vi "CRYO_MASTER_FULL_RUN2.vi"() -> ()   [LabVIEW 2017]
uses:
  LSI218Data.lvclass
  LSI336Data.lvclass
  USBData.lvclass
  6240AData.lvclass
  DMMsData.lvclass
  <vilib>/DAQmx/miscellaneous.llb/DAQmx Fill In Error Info.vi
  <vilib>/DAQmx/create/channels.llb/DAQmx Create Channel (DO-Digital Output).vi
  <vilib>/DAQmx/create/channels.llb/DAQmx Create Channel (AO-Voltage-Basic).vi
  <vilib>/express/express arith-compare/Formula/XNode/ExpressFormulaBlockNode.xnode
  <vilib>/Analysis/NI_AALBase.lvlib
  istr.lib/Agilent 33XXX Series/Agilent 33XXX Series.lvlib
panel:
  in  "Automatic \nScreenshots?":bool=TRUE
  in  "Frontpanel screenshots":bool
  in  "Screenshots interval":i64=3605
  in  "Record interval":i64=10
  out "Cycle #":u32=5047
  in  "Measurement Interval (s)":dbl=1.0
  in  "Stop Button":bool
  in  "?":T1(tab)=enum."LSI CONFIG"
  out "RUN Identifier":string="20210201_135757_RUN_III"
  in  "Base Path (screenshots)":path=path "C:/LabVIEW/DATA/Google/TUCAN Experiments/KEK_cryotests_2019-2020/data/screenshots"
  out "error out (USB6210/6218 AOUT)":errorcluster
  in  "AOUT Labels":string[](array[string])=["PWR400H_I", "PMC183A_I"]
  in  "DOUT Labels":string[](array[string])=["D_V1_NO", "D_V2_NC", "D_CV1", "D_H1"]
  in  "AOUT assignment":tag[](array[tag])=["Dev1/ao0", "Dev1/ao1"]
  out "AO task out":refnum<k21>="20210201_135757_RUN_III_AO"
  in  "Analog Out ON?":bool=TRUE
  in  "InstName (USB6218)":string="USB6218"
  in  "USB6218 Config":T2(array[cluster])=[{"Label"="F_1", "FileFormat"="%5.5f", "Active?"=TRUE, "Physical CH"="Dev1/ai0", " terminal\n type"=10083, "ConversionType"={"Type"=enum."SimpleProp", "ConversionParameters"=[0.0, 5.0, 0.0, 500.0]}, "VoltageLimits"=[0.0, 5.0]}, {"Label"="F_2", "FileFormat"="%5.5f", "Active?"=TRUE, "Physical CH"="Dev1/ai1", " terminal\n type"=10083, "ConversionType"={"Type"=enum."SimpleProp", "ConversionParameters"=[0.0, 5.0, 0.0, 200.0]}, "VoltageLimits"=[0.0, 5.0]}, {"Label"="F_3", "FileFormat"="%5.5f", "Active?"=TRUE, "Physical CH"="Dev1/ai2", " terminal\n type"=10083, "ConversionType"={"Type"=enum."SimpleProp", "ConversionParameters"=[0.0, 5.0, 0.0, 200.0]}, "VoltageLimits"=[0.0, 5.0]}, {"Label"="F_4", "FileFormat"="%5.5f", "Active?"=TRUE, "Physical CH"="Dev1/ai3", " terminal\n type"=10083, "ConversionType"={"Type"=enum."SimpleProp", "ConversionParameters"=[0.0, 5.0, 0.0, 500.0]}, "VoltageLimits"=[0.0, 5.0]}, {"Label"="F_5", "FileFormat"="%5.5f", "Active?"=TRUE, "Physical CH"="Dev1/ai4", " terminal\n type"=10083, "ConversionType"={"Type"=enum."SimpleProp", "ConversionParameters"=[0.0, 5.0, 0.0, 500.0]}, "VoltageLimits"=[0.0, 5.0]}, {"Label"="I_CV", "FileFormat"="%3.5f", "Active?"=TRUE, "Physical CH"="Dev1/ai5", " terminal\n type"=10083, "ConversionType"={"Type"=enum."Raw", "ConversionParameters"=[0.0, 0.0, 0.0, 0.0]}, "VoltageLimits"=[0.0, 10.0]}, {"Label"="CV1_answer", "FileFormat"="%3.5f", "Active?"=TRUE, "Physical CH"="Dev1/ai6", " terminal\n type"=10083, "ConversionType"={"Type"=enum."SimpleProp", "ConversionParameters"=[1.0, 5.0, 0.0, 100.0]}, "VoltageLimits"=[0.0, 5.0]}, {"Label"="P_Dewar", "FileFormat"="%5.5e", "Active?"=TRUE, "Physical CH"="Dev1/ai7", " terminal\n type"=10083, "ConversionType"={"Type"=enum."SimpleProp", "ConversionParameters"=[1.0, 5.0, 0.0, 200000.0]}, "VoltageLimits"=[0.0, 5.0]}] {"terminal\n type" items=["Default"=-1, "RSE"=10083, "NRSE"=10078, "Differential"=10106, "Pseudodifferential"=12529]}
  out "error out (USB6218)":errorcluster
  out "error out (USB6210/6218 DOUT)":errorcluster
  out "DOUT task out":refnum<k21>="20210201_135757_DO"
  in  "DOUT Physical CH":tag[](array[tag])=["Dev1/port1/line0", "Dev1/port1/line1", "Dev1/port1/line2", "Dev1/port1/line3"]
  in  "Digital Out ON?":bool=TRUE
  in  "USB6210 Config":T2(array[cluster])=[{"Label"="P_ins", "FileFormat"="%5.5e", "Active?"=TRUE, "Physical CH"="Dev2/ai0", " terminal\n type"=10083, "ConversionType"={"Type"=enum."CC-10_LOG", "ConversionParameters"=[0.5, 9.0, 0.0, 1.0]}, "VoltageLimits"=[0.0, 10.0]}, {"Label"="P_4Kres", "FileFormat"="%5.5e", "Active?"=TRUE, "Physical CH"="Dev2/ai1", " terminal\n type"=10083, "ConversionType"={"Type"=enum."SimpleProp", "ConversionParameters"=[1.0, 5.0, 0.0, 200000.0]}, "VoltageLimits"=[0.0, 5.0]}, {"Label"="P_3HeIN", "FileFormat"="%5.5e", "Active?"=TRUE, "Physical CH"="Dev2/ai2", " terminal\n type"=10083, "ConversionType"={"Type"=enum."SimpleProp", "ConversionParameters"=[1.0, 5.0, 0.0, 200000.0]}, "VoltageLimits"=[0.0, 5.0]}, {"Label"="P_SldRTN", "FileFormat"="%5.5e", "Active?"=TRUE, "Physical CH"="Dev2/ai3", " terminal\n type"=10083, "ConversionType"={"Type"=enum."SimpleProp", "ConversionParameters"=[1.0, 5.0, 0.0, 200000.0]}, "VoltageLimits"=[0.0, 5.0]}, {"Label"="P_3Hepot", "FileFormat"="%5.5e", "Active?"=TRUE, "Physical CH"="Dev2/ai4", " terminal\n type"=10083, "ConversionType"={"Type"=enum."SimpleProp", "ConversionParameters"=[0.0, 10.0, 0.0, 133320.0]}, "VoltageLimits"=[0.0, 10.0]}, {"Label"="P_1Kpot", "FileFormat"="%5.5e", "Active?"=TRUE, "Physical CH"="Dev2/ai5", " terminal\n type"=10083, "ConversionType"={"Type"=enum."SimpleProp", "ConversionParameters"=[0.0, 10.0, 0.0, 133320.0]}, "VoltageLimits"=[0.0, 10.0]}, {"Label"="P_Dewar(old)", "FileFormat"="%5.5e", "Active?"=FALSE, "Physical CH"="Dev2/ai6", " terminal\n type"=10083, "ConversionType"={"Type"=enum."SimpleProp", "ConversionParameters"=[1.0, 5.0, 0.0, 200000.0]}, "VoltageLimits"=[0.0, 5.0]}, {"Label"="DP_HEX4", "FileFormat"="%5.5e", "Active?"=TRUE, "Physical CH"="Dev2/ai7", " terminal\n type"=10083, "ConversionType"={"Type"=enum."SimpleProp", "ConversionParameters"=[1.0, 5.0, 0.0, 1000.0]}, "VoltageLimits"=[0.0, 5.0]}, {"Label"="DP_HEX5", "FileFormat"="%5.5e", "Active?"=TRUE, "Physical CH"="Dev2/ai8", " terminal\n type"=10083, "ConversionType"={"Type"=enum."SimpleProp", "ConversionParameters"=[1.0, 5.0, 0.0, 1000.0]}, "VoltageLimits"=[0.0, 5.0]}, {"Label"="L1", "FileFormat"="%5.5f", "Active?"=TRUE, "Physical CH"="Dev2/ai9", " terminal\n type"=10083, "ConversionType"={"Type"=enum."SimpleProp", "ConversionParameters"=[0.0, 10.0, 0.0, 100.0]}, "VoltageLimits"=[0.0, 10.0]}, {"Label"="L2-1", "FileFormat"="%5.5f", "Active?"=TRUE, "Physical CH"="Dev2/ai10", " terminal\n type"=10083, "ConversionType"={"Type"=enum."SimpleProp", "ConversionParameters"=[0.0, 10.0, 0.0, 100.0]}, "VoltageLimits"=[0.0, 10.0]}, {"Label"="L2-2", "FileFormat"="%5.5f", "Active?"=TRUE, "Physical CH"="Dev2/ai11", " terminal\n type"=10083, "ConversionType"={"Type"=enum."SimpleProp", "ConversionParameters"=[0.0, 10.0, 0.0, 100.0]}, "VoltageLimits"=[0.0, 10.0]}, {"Label"="L3", "FileFormat"="%5.5f", "Active?"=TRUE, "Physical CH"="Dev2/ai12", " terminal\n type"=10083, "ConversionType"={"Type"=enum."SimpleProp", "ConversionParameters"=[0.0, 10.0, 0.0, 100.0]}, "VoltageLimits"=[0.0, 10.0]}, {"Label"="P_HEX7OUT", "FileFormat"="%5.5e", "Active?"=TRUE, "Physical CH"="Dev2/ai13", " terminal\n type"=10083, "ConversionType"={"Type"=enum."SimpleProp", "ConversionParameters"=[1.0, 5.0, 0.0, 200000.0]}, "VoltageLimits"=[0.0, 5.0]}, {"Label"="P_IP", "FileFormat"="%5.5e", "Active?"=TRUE, "Physical CH"="Dev2/ai14", " terminal\n type"=10083, "ConversionType"={"Type"=enum."CC-10_LOG", "ConversionParameters"=[0.5, 9.0, 0.0, 1.0]}, "VoltageLimits"=[0.0, 10.0]}, {"Label"="V_H1", "FileFormat"="%3.5f", "Active?"=TRUE, "Physical CH"="Dev2/ai15", " terminal\n type"=10083, "ConversionType"={"Type"=enum."Raw", "ConversionParameters"=[0.0, 1.0, 0.0, 1.0]}, "VoltageLimits"=[0.0, 10.0]}] {"terminal\n type" items=["Default"=-1, "RSE"=10083, "NRSE"=10078, "Differential"=10106, "Pseudodifferential"=12529]}
  in  "RUN label":string="RUN_III"
  in  "Base Path":path=path "C:/LabVIEW/DATA/RUN_3"
  in  "InstName (USB6210)":string="USB6210"
  out "error out (USB6210)":errorcluster
  out "File Refn USB AO":refnum<file>
  out "File Refn USB DO":refnum<file>
  out "error out (LSI336)":errorcluster
  in  "InstName (LSI336)":string="LSI336"
  in  "FileFormat (336)":string="%4.4f"
  in  "LSI336Settings(X,Y)":T3(array[cluster])=[{"LSIName"="LSi336X", "Labels"=["T1K3-1", "T1K3-2", "T3He5", "T3He8"], "SensorLocations"=[enum."T1K3-1", enum."T1K3-2", enum."T3He5", enum."T3He8"], "Active?"=TRUE, "VISA res. name"="COM15_LSI336Y"}, {"LSIName"="LSi336Y", "Labels"=["T3He6-1", "T3He6-2", "T3He7-1", "T3He7-2"], "SensorLocations"=[enum."T3He6-1", enum."T3He6-2", enum."T3He7-1", enum."T3He7-2"], "Active?"=TRUE, "VISA res. name"="COM20_LSI336X"}]
  in  "FileFormat (218)":string="%4.4f"
  in  "InstName (LSI218)":string="LSI218"
  in  "LSI218Settings(A-F)":T3(array[cluster])=[{"LSIName"="LSI218A", "Labels"=["T3He10", "T3He1-1", "TTH3", "TTH4", "TTH1", "TTH2", "T4He1", "T1K1"], "SensorLocations"=[enum."T3He10", enum."T3He1-1", enum."TTH3", enum."TTH4", enum."TTH1", enum."TTH2", enum."T4He1", enum."T1K1"], "Active?"=TRUE, "VISA res. name"="GPIB0::7::INSTR"}, {"LSIName"="LSI218B", "Labels"=["N.C.", "N.C.", "N.C.", "N.C.", "T3He2-1", "T3He2-2", "T3He3", "T3He1-4"], "SensorLocations"=[enum."N.C.", enum."N.C.", enum."N.C.", enum."N.C.", enum."T3He2-1", enum."T3He2-2", enum."T3He3", enum."T3He1-4"], "Active?"=TRUE, "VISA res. name"="GPIB0::4::INSTR"}, {"LSIName"="LSI218C", "Labels"=["T4He3-1", "T4He3-2", "T4He3-3", "T4He3-4", "T4He2-1", "T4He2-2", "T4He4", "T4He5"], "SensorLocations"=[enum."T4He3-1", enum."T4He3-2", enum."T4He3-3", enum."T4He3-4", enum."T4He2-1", enum."T4He2-2", enum."T4He4", enum."T4He5"], "Active?"=TRUE, "VISA res. name"="GPIB0::3::INSTR"}, {"LSIName"="LSI218D", "Labels"=["T4He6", "T4He9", "T3He1-2", "T3He1-3", "T4He7", "T4He8", "T4He10", "T1K6"], "SensorLocations"=[enum."T4He6", enum."T4He9", enum."T3He1-2", enum."T3He1-3", enum."T4He7", enum."T4He8", enum."T4He10", enum."T1K6"], "Active?"=TRUE, "VISA res. name"="GPIB0::5::INSTR"}, {"LSIName"="LSI218E", "Labels"=["TIP1", "N.C.", "TIP2", "N.C.", "TIP3", "TIP4", "TIP5", "N.C."], "SensorLocations"=[enum."TIP1", enum."N.C.", enum."TIP2", enum."N.C.", enum."TIP3", enum."TIP4", enum."TIP5", enum."N.C."], "Active?"=TRUE, "VISA res. name"="GPIB0::11::INSTR"}, {"LSIName"="LSI218F", "Labels"=["T1K2", "T1K4", "T1K5", "T3He4", "T3He9", "TIP6", "N.C.", "N.C."], "SensorLocations"=[enum."T1K2", enum."T1K4", enum."T1K5", enum."T3He4", enum."T3He9", enum."TIP6", enum."N.C.", enum."N.C."], "Active?"=TRUE, "VISA res. name"="GPIB0::8::INSTR"}]
  out "error out (LSI218)":errorcluster
  out "RUN Identifier 2":string="20210201_135757_RUN_III" caption="RUN Identifier"
  out "Graph 3":T4(graph) caption="XY Graph"
  out "Graph 1":T4(graph) caption="XY Graph"
  in  "FIle suffix 4":string="Graph4_noise"
  in  "Take Screenshot! 4":bool
  in  "Take Screenshot! 3":bool
  in  "Take Screenshot! 2":bool
  in  "Take Screenshot! 1":bool
  in  "FIle suffix 3":string="Graph3_noise"
  in  "FIle suffix 2":string="Graph2_noise"
  in  "FIle suffix 1":string="Graph1_noise"
  in  "log/linear 2":bool
  in  "Tab Control 2":T5(tab)=enum."Temperature (3)"
  in  "Plot selecter (USB6210)\n    1      2     3     4":bool[][](array[boolean])=[[TRUE, FALSE, FALSE, FALSE], [TRUE, FALSE, FALSE, FALSE], [TRUE, FALSE, FALSE, FALSE], [TRUE, FALSE, FALSE, FALSE], [TRUE, FALSE, FALSE, FALSE], [TRUE, FALSE, FALSE, FALSE], [TRUE, FALSE, FALSE, FALSE], [FALSE, TRUE, FALSE, FALSE], [FALSE, TRUE, FALSE, FALSE], [FALSE, TRUE, FALSE, FALSE], [FALSE, TRUE, FALSE, FALSE], [FALSE, TRUE, FALSE, FALSE], [FALSE, TRUE, FALSE, FALSE], [TRUE, FALSE, FALSE, FALSE], [TRUE, FALSE, FALSE, FALSE], [FALSE, FALSE, FALSE, FALSE]]
  out "All Labels (USB6210)":string[](array[string])=["P_ins", "P_4Kres", "P_3HeIN", "P_SldRTN", "P_3Hepot", "P_1Kpot", "P_Dewar(old)", "DP_HEX4", "DP_HEX5", "L1", "L2-1", "L2-2", "L3", "P_HEX7OUT", "P_IP", "V_H1"]
  out "Last Data \n(USB6210)":dbl[](array[numeric])=[0.0022537913465804096, 117802.86707498573, 116158.43504093104, 117235.53795122683, 102003.2967982825, 102347.86616711758, 0.0, -47.76057639593803, -0.7635102043834219, 0.14875711111916923, 0.03761845613593001, 0.017232075569376254, 99.40279540247681, 116669.85333759272, 0.0006269205762310876, 5.814560646237538] format="%#_6e"
  out "Time of Last Measurement (USB6210)":timestamp=timestamp(3695005369.6779566 s since 1904-01-01)
  out "USB6210 Status":T6(ring)=enum."Ready"
  out "Last Vol\n(USB6210)":dbl[](array[numeric])=[6.176456853542879, 3.3560573414997146, 3.323168700818621, 3.3447107590245366, 7.651012361107298, 7.676857648298649, 0.0, 0.8089576944162479, 0.9969459591824663, 0.014875711111916923, 0.0037618456135930013, 0.0017232075569376254, 9.940279540247682, 3.3333970667518544, 5.898606262050578, 5.814560646237538] format="%_5f"
  out "Time of Last Measurement (USB6218)":timestamp=timestamp(3695005369.684819 s since 1904-01-01)
  out "USB6218 Status":T6(ring)=enum."Ready"
  out "Last Vol \n(USB6218)":dbl[](array[numeric])=[0.33539560717986167, 0.0011817571226759374, 0.006179348059626015, 0.231991528158746, 1.5216321927785632, -0.07609488128103897, 0.0006228160374054145, 3.4048662521971877] format="%_5f"
  out "Last Data \n(USB6218)":dbl[](array[numeric])=[33.53956071798617, 0.047270284907037496, 0.2471739223850406, 23.199152815874598, 152.1632192778563, -0.07609488128103897, -24.984429599064864, 120243.3126098594] format="%#_6e"
  out "All Labels (USB6218)":string[](array[string])=["F_1", "F_2", "F_3", "F_4", "F_5", "I_CV", "CV1_answer", "P_Dewar"]
  in  "Plot selecter (USB6218)\n    1      2     3     4":bool[][](array[boolean])=[[FALSE, FALSE, TRUE, FALSE], [FALSE, FALSE, TRUE, FALSE], [FALSE, FALSE, TRUE, FALSE], [FALSE, FALSE, TRUE, FALSE], [FALSE, FALSE, TRUE, FALSE], [FALSE, FALSE, TRUE, FALSE], [FALSE, FALSE, FALSE, FALSE], [TRUE, FALSE, FALSE, FALSE], [FALSE, FALSE, TRUE, FALSE], [FALSE, FALSE, FALSE, TRUE], [FALSE, FALSE, FALSE, TRUE], [FALSE, FALSE, FALSE, TRUE], [FALSE, FALSE, FALSE, TRUE], [FALSE, FALSE, FALSE, FALSE], [FALSE, FALSE, FALSE, FALSE], [FALSE, FALSE, FALSE, FALSE]]
  out "Time of Last Measurement (LSI218)":timestamp=timestamp(3695005369.6769576 s since 1904-01-01)
  out "LSI218 Status":T7(ring)=enum."Measuring"
  out "Last Data \nLSI218 (1)":dbl[](array[numeric])=[292.38, 292.73, 294.52, 295.87, 285.32, 295.14, 162.92, 163.07, 30.0, 0.0, 0.0, 0.0, 289.67, 288.5, 171.24, 292.17, 292.49, 292.62, 292.39, 292.29, 262.97, 263.24, 294.16, 294.29]
  out "Labels LSI218 (1)":string[](array[string])=["T3He10", "T3He1-1", "TTH3", "TTH4", "TTH1", "TTH2", "T4He1", "T1K1", "N.C.", "N.C.", "N.C.", "N.C.", "T3He2-1", "T3He2-2", "T3He3", "T3He1-4", "T4He3-1", "T4He3-2", "T4He3-3", "T4He3-4", "T4He2-1", "T4He2-2", "T4He4", "T4He5"]
  in  "Plot selecter LSI218(1)\n    1      2     3     4":bool[][](array[boolean])=[[FALSE, FALSE, FALSE, TRUE], [FALSE, FALSE, FALSE, TRUE], [FALSE, TRUE, FALSE, TRUE], [FALSE, TRUE, FALSE, TRUE], [FALSE, TRUE, FALSE, TRUE], [FALSE, TRUE, FALSE, TRUE], [FALSE, FALSE, FALSE, TRUE], [FALSE, FALSE, FALSE, TRUE], [FALSE, FALSE, FALSE, FALSE], [FALSE, FALSE, FALSE, FALSE], [FALSE, FALSE, FALSE, FALSE], [FALSE, FALSE, FALSE, FALSE], [FALSE, FALSE, FALSE, TRUE], [FALSE, FALSE, FALSE, TRUE], [FALSE, FALSE, FALSE, TRUE], [FALSE, FALSE, FALSE, TRUE], [FALSE, FALSE, FALSE, TRUE], [FALSE, FALSE, FALSE, TRUE], [FALSE, FALSE, FALSE, TRUE], [FALSE, FALSE, FALSE, TRUE], [FALSE, FALSE, FALSE, TRUE], [FALSE, FALSE, FALSE, TRUE], [FALSE, FALSE, FALSE, TRUE], [FALSE, FALSE, FALSE, TRUE]]
  out "Active?\n (1)":bool[](array[boolean])=[TRUE, TRUE, TRUE, TRUE, TRUE, TRUE, TRUE, TRUE, TRUE, TRUE, TRUE, TRUE, TRUE, TRUE, TRUE, TRUE, TRUE, TRUE, TRUE, TRUE, TRUE, TRUE, TRUE, TRUE]
  out "Labels LSI218 (2)":string[](array[string])=["T4He6", "T4He9", "T3He1-2", "T3He1-3", "T4He7", "T4He8", "T4He10", "T1K6", "TIP1", "N.C.", "TIP2", "N.C.", "TIP3", "TIP4", "TIP5", "N.C.", "T1K2", "T1K4", "T1K5", "T3He4", "T3He9", "TIP6", "N.C.", "N.C."]
  out "Active?\n(2)":bool[](array[boolean])=[TRUE, TRUE, TRUE, TRUE, TRUE, TRUE, TRUE, TRUE, TRUE, TRUE, TRUE, TRUE, TRUE, TRUE, TRUE, TRUE, TRUE, TRUE, TRUE, TRUE, TRUE, TRUE, TRUE, TRUE]
  out "Last Data \nLSI218 (2)":dbl[](array[numeric])=[294.69, 295.53, 292.84, 292.58, 294.67, 293.86, 293.89, 292.4, 293.56, 0.0, 294.5, 688.49, 293.25, 285.52, 294.89, 688.58, 281.54, 266.94, 289.77, 294.88, 232.7, 292.33, 0.433, 0.0]
  in  "Plot selecter LSI218(2)\n    1      2     3     4":bool[][](array[boolean])=[[FALSE, FALSE, FALSE, TRUE], [FALSE, FALSE, FALSE, TRUE], [FALSE, FALSE, FALSE, TRUE], [FALSE, FALSE, FALSE, TRUE], [FALSE, FALSE, FALSE, TRUE], [FALSE, FALSE, FALSE, TRUE], [FALSE, FALSE, FALSE, TRUE], [FALSE, FALSE, FALSE, FALSE], [FALSE, FALSE, FALSE, FALSE], [FALSE, FALSE, FALSE, FALSE], [FALSE, FALSE, FALSE, FALSE], [FALSE, FALSE, FALSE, FALSE], [FALSE, FALSE, FALSE, FALSE], [FALSE, FALSE, FALSE, FALSE], [FALSE, FALSE, FALSE, FALSE], [FALSE, FALSE, FALSE, FALSE], [FALSE, FALSE, FALSE, TRUE], [FALSE, FALSE, FALSE, TRUE], [FALSE, FALSE, FALSE, TRUE], [FALSE, FALSE, FALSE, TRUE], [FALSE, FALSE, FALSE, FALSE], [FALSE, FALSE, FALSE, FALSE], [FALSE, FALSE, FALSE, FALSE], [FALSE, FALSE, FALSE, FALSE]]
  in  "Plot selecter LSI336 \n     1      2     3     4":bool[][](array[boolean])=[[FALSE, FALSE, FALSE, TRUE], [FALSE, FALSE, FALSE, TRUE], [FALSE, FALSE, FALSE, TRUE], [FALSE, FALSE, FALSE, TRUE], [FALSE, FALSE, FALSE, TRUE], [FALSE, FALSE, FALSE, TRUE], [FALSE, FALSE, FALSE, TRUE], [FALSE, FALSE, FALSE, TRUE]]
  out "Time of Last Measurement (LSI336)":timestamp=timestamp(3695005369.6769576 s since 1904-01-01)
  out "Last Data \nLSI336":dbl[](array[numeric])=[253.479, 282.867, 281.926, 273.202, 241.683, 239.413, 247.474, 294.303]
  out "Active?\n(LSI336)":bool[](array[boolean])=[TRUE, TRUE, TRUE, TRUE, TRUE, TRUE, TRUE, TRUE]
  out "Labels LSI336":string[](array[string])=["T1K3-1", "T1K3-2", "T3He5", "T3He8", "T3He6-1", "T3He6-2", "T3He7-1", "T3He7-2"]
  out "LSI336 Status":T7(ring)=enum."Measuring"
  in  "log/linear 1":bool
  out "Graph 2":T4(graph) caption="XY Graph"
  out "Graph 4":T4(graph) caption="XY Graph"
  in  "log/linear 4":bool
  in  "log/linear 3":bool
  out "RUN Identifier 3":string="20210201_135757_RUN_III" caption="RUN Identifier"
  in  "AutoFill Source (P)":T8(ring)=enum."USB6218AI"
  in  "AutoFill Source (L)":T8(ring)
  out "RUN Identifier 4":string="20210201_135757_RUN_III" caption="RUN Identifier"
  out "Fill (false)":bool
  in  "Fill state":bool=TRUE
  out "state 1 (false)":bool
  out "state 1":bool=TRUE
  out "state 2":bool
  out "state 2 (false)":bool=TRUE
  out "Status V2 CTRL":enum16{"Pressurize", "Release"}(ring)=enum."Release"
  out "Status V1 CTRL":enum16{"Pressurize", "Release"}(ring)
  out "Lav (%)":dbl=99.41665308336506 format="%0.2f"
  out "Lstd":dbl=0.013434980613335595 format="%0.2f"
  out "Last N M.A. Levels":dbl[](array[numeric])=[99.41430432174354, 99.41430432174258, 99.41726375820552, 99.40937192771227, 99.40739897018216, 99.4064124913516, 99.40443953372208, 99.41397549556436, 99.41430432175262, 99.41545521369594, 99.41430432178369, 99.40772779639909, 99.44899551077012, 99.44488518248531] format="%_5e"
  out "Lstd history":dbl(graph)=0.010699490860246581
  out "Lav history":dbl(graph)=99.41445699237359
  out "Target Index (L)":i32=12
  in  "Auto Fll He L. label":string="L3"
  out "Target Index (P)":i32=7
  in  "Auto Fll Dewar P. label":string="P_Dewar"
  out "He Level":T9(graph)=[{"TimeArray"=[timestamp(3695005356.559472 s since 1904-01-01), timestamp(3695005357.5598545 s since 1904-01-01), timestamp(3695005358.560987 s since 1904-01-01), timestamp(3695005359.5608015 s since 1904-01-01), timestamp(3695005360.560333 s since 1904-01-01), timestamp(3695005361.562082 s since 1904-01-01), timestamp(3695005362.560125 s since 1904-01-01), timestamp(3695005363.562583 s since 1904-01-01), timestamp(3695005364.5623016 s since 1904-01-01), timestamp(3695005365.5639224 s since 1904-01-01), timestamp(3695005366.5634737 s since 1904-01-01), timestamp(3695005367.56578 s since 1904-01-01), timestamp(3695005368.6749086 s since 1904-01-01), timestamp(3695005369.6779566 s since 1904-01-01)], "Filtered X"=[99.41331784290249, 99.4139754955639, 99.41594845308731, 99.39424591929536, 99.40542601278204, 99.41002958024174, 99.40805662256918, 99.4323897666645, 99.4067413175351, 99.41463314801497, 99.40345305492019, 99.40608366512608, 99.57181217501929, 99.39819183487565]}, {"TimeArray"=[timestamp(3695005356.559472 s since 1904-01-01), timestamp(3695005357.5598545 s since 1904-01-01), timestamp(3695005358.560987 s since 1904-01-01), timestamp(3695005359.5608015 s since 1904-01-01), timestamp(3695005360.560333 s since 1904-01-01), timestamp(3695005361.562082 s since 1904-01-01), timestamp(3695005362.560125 s since 1904-01-01), timestamp(3695005363.562583 s since 1904-01-01), timestamp(3695005364.5623016 s since 1904-01-01), timestamp(3695005365.5639224 s since 1904-01-01), timestamp(3695005366.5634737 s since 1904-01-01), timestamp(3695005367.56578 s since 1904-01-01), timestamp(3695005368.6749086 s since 1904-01-01), timestamp(3695005369.6779566 s since 1904-01-01)], "Filtered X"=[99.41430432174354, 99.41430432174258, 99.41726375820552, 99.40937192771227, 99.40739897018216, 99.4064124913516, 99.40443953372208, 99.41397549556436, 99.41430432175262, 99.41545521369594, 99.41430432178369, 99.40772779639909, 99.44899551077012, 99.44488518248531]}] caption="XY Graph"
  in  "P_safelimit_high (Pa)":dbl=300000.0 format="%_4e"
  in  "P_safelimit_low (Pa)":dbl=100.0 format="%_4e"
  in  "Auto Fill ON?":bool=TRUE
  out "Pstd history":dbl(graph)=75.26521633475697
  out "Pav history":dbl(graph)=120829.26024406902
  in  "Mov. Avg Interval":i64=4
  in  "V2 (N.C.)":bool
  in  "V1 (N.O.)":bool
  in  "N for sampling":i64=7
  in  "L_low (%)":dbl=100.0 format="%_3f"
  in  "L_high (%)":dbl=100.0 format="%_3g"
  in  "P_2_low (Pa)":dbl=115000.0 format="%_4e"
  in  "P_1_low (Pa)":dbl=120000.0 format="%_4g"
  in  "P_2_high (Pa)":dbl=120000.0 format="%_4e"
  in  "P_1_high (Pa)":dbl=140000.0 format="%_4e"
  out "Dewar Pressure":T9(graph)=[{"TimeArray"=[timestamp(3695005356.559472 s since 1904-01-01), timestamp(3695005357.5598545 s since 1904-01-01), timestamp(3695005358.560987 s since 1904-01-01), timestamp(3695005359.5608015 s since 1904-01-01), timestamp(3695005360.560333 s since 1904-01-01), timestamp(3695005361.562082 s since 1904-01-01), timestamp(3695005362.560125 s since 1904-01-01), timestamp(3695005363.562583 s since 1904-01-01), timestamp(3695005364.5623016 s since 1904-01-01), timestamp(3695005365.5639224 s since 1904-01-01), timestamp(3695005366.5634737 s since 1904-01-01), timestamp(3695005367.56578 s since 1904-01-01), timestamp(3695005368.6749086 s since 1904-01-01), timestamp(3695005369.6779566 s since 1904-01-01)], "Filtered X"=[120596.75998069301, 120853.21481684512, 121149.12424242542, 120609.911510447, 120718.41163365253, 120774.30563686597, 120581.96450945176, 120978.1543516866, 120989.66194088905, 120800.60869664834, 121071.85900376887, 120756.22228285341, 120943.63158576176, 120891.02546541338]}, {"TimeArray"=[timestamp(3695005356.559472 s since 1904-01-01), timestamp(3695005357.5598545 s since 1904-01-01), timestamp(3695005358.560987 s since 1904-01-01), timestamp(3695005359.5608015 s since 1904-01-01), timestamp(3695005360.560333 s since 1904-01-01), timestamp(3695005361.562082 s since 1904-01-01), timestamp(3695005362.560125 s since 1904-01-01), timestamp(3695005363.562583 s since 1904-01-01), timestamp(3695005364.5623016 s since 1904-01-01), timestamp(3695005365.5639224 s since 1904-01-01), timestamp(3695005366.5634737 s since 1904-01-01), timestamp(3695005367.56578 s since 1904-01-01), timestamp(3695005368.6749086 s since 1904-01-01), timestamp(3695005369.6779566 s since 1904-01-01)], "Filtered X"=[120840.88525717883, 120738.13892881335, 120806.77347609057, 120802.25263760264, 120832.66555084252, 120812.93825584772, 120671.14832260432, 120763.20903291422, 120831.02160972334, 120837.59737466894, 120960.07099824822, 120904.58798103992, 120893.0803922581, 120915.68458444934]}] caption="XY Graph"
  out "Last N M.A. Pressures":dbl[](array[numeric])=[120840.88525717883, 120738.13892881335, 120806.77347609057, 120802.25263760264, 120832.66555084252, 120812.93825584772, 120671.14832260432, 120763.20903291422, 120831.02160972334, 120837.59737466894, 120960.07099824822, 120904.58798103992, 120893.0803922581, 120915.68458444934] format="%_5e"
  out "Pav (Pa)":dbl=120829.289600163 format="%0.4e"
  out "Pstd":dbl=75.30141666084926 format="%0.4e"
  out "File Refn DewarCTRL":refnum<file>
  out "Error Out (Dewar CTRL":errorcluster
  in  "lower limit (mA) \n(PMC)":dbl=4.0 format="%_3f"
  in  "upper limit (mA)\n (PMC)":dbl=40.0 format="%_3f"
  in  "OUTPUT\n(PMC)":bool
  in  "Set Current (mA)\n (PMC)":dbl=4.0 min=4.0 max=40.0 format="%_3g"
  in  "update values":bool
  out "Monitor Current (mA)":dbl=2.210431911345124 min=0.0 max=1.9 format="%_4e"
  in  "update current":bool
  out "USB 6218 AOUT":dbl[](array[numeric])=[0.02, 0.004, 0.1491827711262358, 0.06969546425555169]
  out "Graph 7":T10(graph) caption="XY Graph"
  in  "lower limit (mA) \n(PWR)":dbl=4.0 format="%_3f"
  in  "upper limit (mA)\n (PWR)":dbl=20.0 format="%_3f"
  in  "lower limit (mA)":dbl=4.0 format="%_3f"
  in  "SetCurrent 2 (mA)":dbl=4.0 min=4.0 max=500.0 format="%_3f"
  in  "upper limit (mA)":dbl=500.0 format="%_3f"
  out "error out (KIKUSI CTRL)":errorcluster
  out "ActualVoltage (V)":dbl[](array[numeric]) format="%_6g"
  out "ActualCurrent (A)":dbl[](array[numeric])=[0.004, 0.004] format="%_3e"
  in  "SetCurrent 1 (mA)":dbl=4.0 min=4.0 max=500.0 format="%_3g"
  in  "Output\n (ADCMT)":bool[](array[boolean])=[FALSE, FALSE]
  out "error out (ADCMT6420A)":errorcluster
  in  "Voltage limits (V)":dbl[](array[numeric])=[12.0, 12.0] format="%_3f"
  in  "CtrlLabels":string[](array[string])=["CV2", "CV3"]
  in  "VISA":refnum<visa-resource-name>[](array[refnum])=["GPIB0::1::INSTR", "GPIB0::12::INSTR"]
  out "Initialized?":bool
  in  "InstName":string="ADCMT6240"
  out "Graph 6":T9(graph)=[{"TimeArray"=[timestamp(3694992537.004159 s since 1904-01-01), timestamp(3694992568.1320286 s since 1904-01-01), timestamp(3694992635.1700454 s since 1904-01-01)], "Filtered X"=[0.004, 0.02, 0.004]}, {"TimeArray"=[timestamp(3694992537.004159 s since 1904-01-01), timestamp(3694992568.1320286 s since 1904-01-01), timestamp(3694992635.1700454 s since 1904-01-01)], "Filtered X"=[0.004, 0.004, 0.004]}, {"TimeArray"=[timestamp(3694992537.004159 s since 1904-01-01), timestamp(3694992568.1320286 s since 1904-01-01), timestamp(3694992635.1700454 s since 1904-01-01)], "Filtered X"=[0.004, 0.02, 0.004]}, {"TimeArray"=[timestamp(3694992537.004159 s since 1904-01-01), timestamp(3694992568.1320286 s since 1904-01-01), timestamp(3694992635.1700454 s since 1904-01-01)], "Filtered X"=[0.004, 0.004, 0.004]}] caption="XY Graph"
  in  "Initialize":bool
  in  "CONTROL KIKUSUI?":bool=TRUE
  in  "OUTPUT\n(PWR)":bool
  in  "Set Current (mA)\n (PWR)":dbl=20.0 min=4.0 max=20.0 format="%_3g"
  out "RUN Identifier 5":string="20210201_135757_RUN_III" caption="RUN Identifier"
  out "ƒ¢T=T_2 -T_1":dbl
  out "Graph DMMs 3":T4(graph) caption="XY Graph"
  out "Q = I *V":dbl
  in  "index I":i64
  in  "index V":i64=1
  out "VariableSources":T11(array[ring])
  in  "DMMsConfig (variables)":T12(array[cluster])=[{"Label"="P_3Hepot", "Active?"=FALSE, "Source"=enum."USB6210", "SourceLabel"="P_3Hepot", "FileFormat"="%6.4e"}, {"Label"="F_1", "Active?"=FALSE, "Source"=enum."USB6218AI", "SourceLabel"="F_1", "FileFormat"="%3.4f"}, {"Label"="F_4", "Active?"=FALSE, "Source"=enum."USB6218AI", "SourceLabel"="F_4", "FileFormat"="%3.4f"}, {"Label"="F_5", "Active?"=FALSE, "Source"=enum."USB6218AI", "SourceLabel"="F_5", "FileFormat"="%3.4f"}, {"Label"="DP_HEX4", "Active?"=FALSE, "Source"=enum."USB6210", "SourceLabel"="DP_HEX4", "FileFormat"="%4.3e"}, {"Label"="T3He6-1", "Active?"=FALSE, "Source"=enum."LSI336", "SourceLabel"="T3He6-1", "FileFormat"="%3.4f"}, {"Label"="T3He6-2", "Active?"=FALSE, "Source"=enum."LSI336", "SourceLabel"="T3He6-2", "FileFormat"="%3.4f"}, {"Label"="T3He7-1", "Active?"=FALSE, "Source"=enum."LSI336", "SourceLabel"="T3He7-1", "FileFormat"="%3.4f"}, {"Label"="T3He7-2", "Active?"=FALSE, "Source"=enum."LSI336", "SourceLabel"="T3He7-2", "FileFormat"="%3.4f"}]
  in  "Measure DMMs?":bool
  out "DMMsLabels":string[](array[string])
  out "Active?":bool[](array[boolean])
  out "DMM LastMeasurements":dbl[](array[numeric])
  out "Graph DMMs 2":T4(graph) caption="XY Graph"
  out "DMMFileName":string
  out "error out (DMMs)":errorcluster={"status"=TRUE, "code"=-1074000000, "source"="ADCMT7351_ADC.lvlib:Error Query.vi<ERR>\nInstrument reports:\n+150,\"Illegal packet received\"\r\n+0,\"No error\"\r\n\n\n\n<b>Complete call chain:</b>\r\n     ADCMT7351_ADC.lvlib:Error Query.vi\r\n     DMMsData.lvclass:DDMs_low_measure.vi\r\n     DMMsData.lvclass:DMMs_measure.vi\r\n     CRYO_MASTER_FULL_dev.vi"}
  out "cycle # (DMMs)":i32=10178
  in  "DMMsConfig":T13(array[cluster])=[{"Label"="I_H2", "Active?"=TRUE, "VISA resource name"="USB0::0x1334::0x0204::262800451::INSTR", "Device"=enum."ADCMT7351", "Measurement"=enum."DC Currents", "FileFormat"="%4.6e"}, {"Label"="V_H2", "Active?"=TRUE, "VISA resource name"="USB0::0x1334::0x0204::262800066::INSTR", "Device"=enum."ADCMT7351", "Measurement"=enum."DC Volts", "FileFormat"="%4.6e"}]
  in  "Measurement Interval DMMs (ms)":i64=500
  in  "InstName DMMs":string="DMMs"
  in  "Initialize (DMMs)":bool
  out "Graph DMMs 1":T4(graph) caption="XY Graph"
  out "error out (DMM graphs)":errorcluster
  in  "Sample #":i32=5
  in  "index T_ 1":i64=6
  in  "index T_2":i64=9
  out "error out (DMMs) 2":errorcluster
  out "P_HEX7OUT":dbl=116643.54242373443 format="%_4e"
  out "P (HEX7 out)":dbl=116643.54242373443 format="%_4e"
  out "DP HEX5":dbl=-2.4572466621291813 format="%_4e"
  out "DP_HEX5":dbl=-2.4572466621291813 format="%_4e"
  in  "Diff pressure HEX5":string="DP_HEX5"
  out "3He pot level":dbl=0.1487571111243332 format="%_4f"
  in  "3He pot":string="L1"
  out "He level (3He)":dbl(slide)=0.1487571111243332 scale=0.0..100.0
  out "He level (1K) b":dbl(slide)=0.01788970075682947 scale=0.0..100.0
  out "He level (1K)":dbl(slide)=0.059320087035186375 scale=0.0..100.0
  out "He level (4K)":dbl(slide)=99.39819183487565 scale=0.0..100.0
  out "1K pot(b1)":dbl=0.01788970075682947 format="%_4f"
  in  "1K pot (b)":string="L2-2"
  in  "1K pot level":string="L2-1"
  out "L(1K) (a1)":dbl=0.059320087035186375 format="%_4f"
  in  "SensorLocation 2":T14(ring)=enum."T3He5"
  out "Temperature 2":dbl=281.936
  out "DP HEX4":dbl=-47.90857270898652 format="%_4e"
  in  "Diff pressure HEX4":string="DP_HEX4"
  out "V2":bool
  out "V1":bool
  out "F5 (3He pump ex.)":dbl=150.52256451261823 format="%_4f"
  out "F4 (3He in to HEX7)":dbl=21.38752641812114 format="%_3f"
  out "F3 (4He rtn flw via HEX7)":dbl=-0.5182465884984702 format="%_4f"
  out "F1 (1K pump exhaust) flow":dbl=32.31646640542272 format="%_4f"
  out "P (Dewar)":dbl=120891.02546541338 format="%_4e"
  out "P (1K pot)":dbl=102359.26413704931 format="%_4e"
  out "P (3He pot)":dbl=102009.43416565923 format="%_4e"
  out "P (shield return)":dbl=117251.98227383036 format="%_4e"
  out "P (3He IN)":dbl=116214.34571877927 format="%_4e"
  out "P (4K reservoir)":dbl=117863.71107164797 format="%_4e"
  out "P (insulation)":dbl=0.0022273278841252572 format="%_4e"
  in  "3He pump exhaust flow":string="F_5"
  out "F_5":dbl=150.52256451261823 format="%_4f"
  in  "3He incoming flow into HEX7":string="F_4"
  out "F_4":dbl=21.38752641812114 format="%_4f"
  out "F_3":dbl=-0.5182465884984702 format="%_4f"
  in  "4He return flow from HEX7":string="F_3"
  out "F_2":dbl=-0.556386098653926 format="%_4f"
  in  "Shield flow":string="F_2"
  out "P_SldRTN":dbl=117251.98227383036 format="%_4e"
  in  "3He pot pressure":string="P_3Hepot"
  out "P_3Hepot":dbl=102009.43416565923 format="%_4e"
  in  "Shield return press.":string="P_SldRTN"
  out "F_1":dbl=32.31646640542272 format="%_4f"
  in  "1K pump exhaust flow":string="F_1"
  out "P_Dewar":dbl=120891.02546541338 format="%_4e"
  in  "Dewar pressure":string="P_Dewar"
  out "P_1Kpot":dbl=102359.26413704931 format="%_4e"
  in  "1Kpot pressure":string="P_1Kpot"
  out "P_3HeIN":dbl=116214.34571877927 format="%_4e"